vi "RX TX Open (N Channel).vi"(0 "resources":T15[](array[numeric]), 1 "option string":string, 3 "direction":T12, 9 "session in":T1[](array[numeric]), 11 "error in":errorcluster, 12 "force download":bool) -> (4 "tx baseband session out":T2[](array[numeric]), 6 "rx baseband session out":T10[](array[numeric]), 10 "session out":T1[](array[numeric]), 15 "error out":errorcluster)   [LabVIEW 2019] (continued)
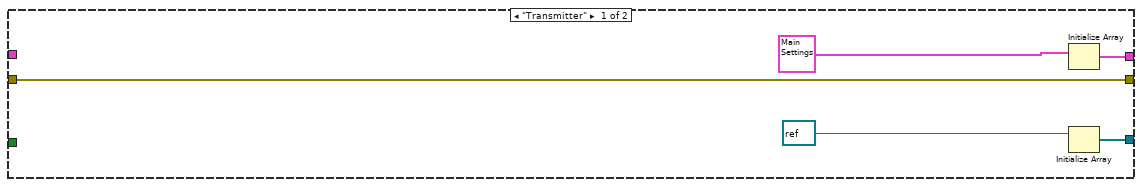
[diagram p2: hidden frame]
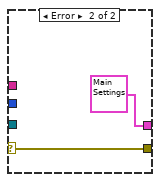
[diagram p4: hidden frame]
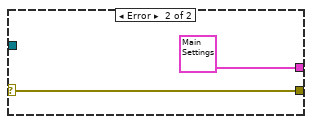
[diagram p5: hidden frame]
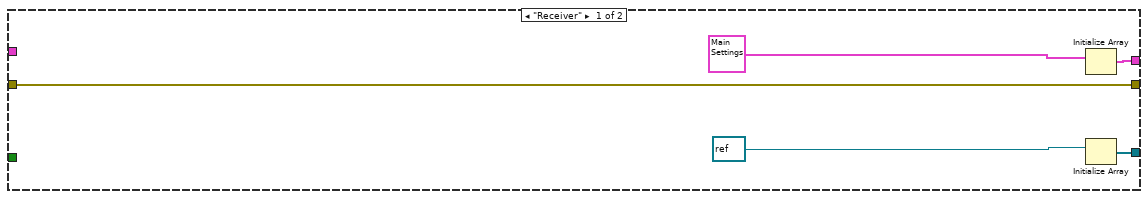
[diagram p6: hidden frame]
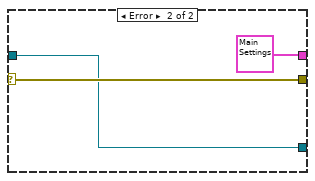
[diagram p7: hidden frame]
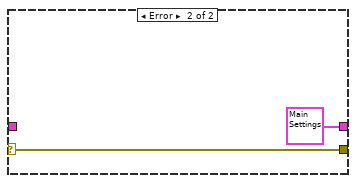
[diagram p10: hidden frame]
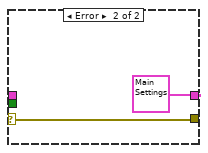
[diagram p12: hidden frame]
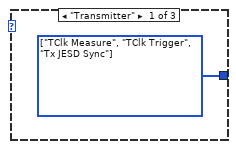
[diagram p13: hidden frame]
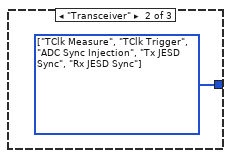
[diagram p14: hidden frame]
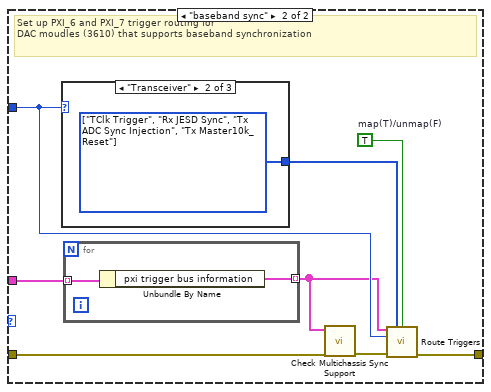
[diagram p15: hidden frame]
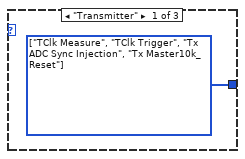
[diagram p16: hidden frame]
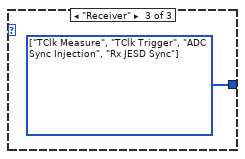
[diagram p17: hidden frame]
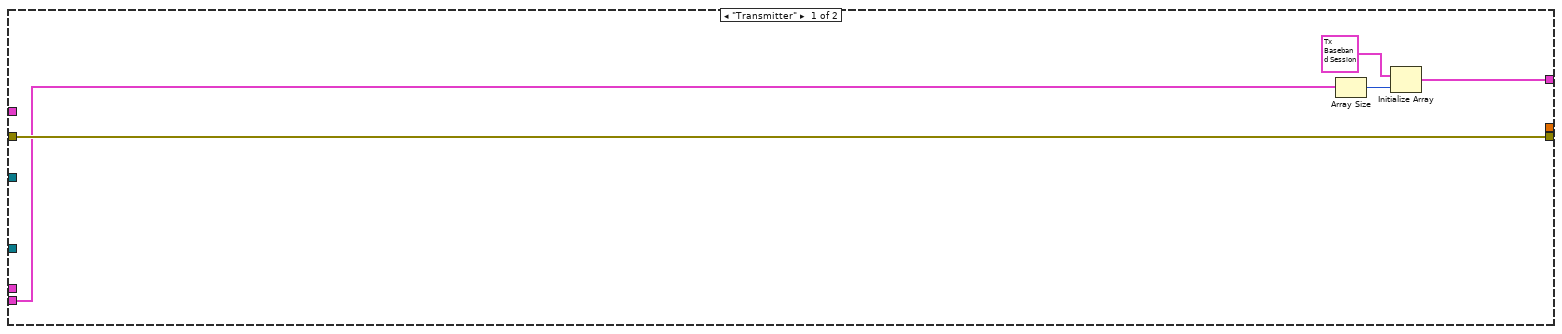
[diagram p18: hidden frame]
          n44 = call "Route Triggers.vi"("pxi trigger bus configuration [channel]"=w230, "route for"=w236, "map(T)/unmap(F)"=w235, "Direction"=w233, "error in"=w231) -> ("error out"=w237:errorcluster)  [unwired: 10 in]
        }
      }
      n45 = case shown="\"Transceiver\", \"Receiver\"" w15 {
        tunnel: w28 -> [w198 w203]
        tunnel: [w197 w202] -> w42
        tunnel: [w198 w201] -> w41
        tunnel: w48 -> [_ w200]
        tunnel: w29 -> [w197 w199]
        frame "Transmitter" {
        }
        frame "Transceiver", "Receiver" {
          n46 = for {
            tunnel: w200 -> [w207]
            shift-right: [w205] -> w202
            shift-left: w199 -> [w208]
            tunnel: w203 -> [w206] mode=indexing
            tunnel: [w204] -> w201 mode=indexing
            # "RX\nInitialize PLL"
            n47 = case shown="No Error" w208 {
              selector: w208 -> [w212 w217]
              tunnel: [w210 w217] -> w205
              tunnel: w206 -> [w213 _]
              tunnel: [w211 T3 {"VISA resource name"=refnum, "Address Space"=0, "window_offset"=0, "register_addresses"={"MM based Registers"={"Revision"=0, "OldestCompatRev"=0, "signature"=0, "scratch"=0, "LedControl"=0, "BoardHwRev"=0, "BoardControl"=0, "ThermalStatus"=0, "BasebandStatus"=0, "BasebandControl"=0, "BasebandAuxSetup"=0, "BasebandAuxStatus"=0, "LmkSyncOutSetup"=0, " AdcSyncOutSetup"=0, " InjSyncOutSetup"=0, " PxiTrig0OutSetup"=0, " PxiTrig1OutSetup"=0, " PxiTrig2OutSetup"=0, " PxiTrig3OutSetup"=0, " PxiTrig4OutSetup"=0, " PxiTrig5OutSetup"=0, " PxiTrig6OutSetup"=0, " PxiTrig7OutSetup"=0}, "CPLD based Registers"={"SlaveSignature"=0, "SlaveRevision"=0, "SlaveOldestCompatRev"=0, "SlaveScratch"=0, "SlaveSetup"=0, "SlaveStatus"=0, "IDacReg_offset"=0, "LMKRegGrp0_offset"=0, "QDacReg_offset"=0, "BrdTempSensorVal"=0, "TempSensorPowerDown"=0, "GPIOReg_offset"=0, "IAdcReg_offset"=0, "QAdcReg_offset"=0, "LMKRegGrp1_offset"=0, "QadcTempSensorVal"=0, "IadcTempSensorVal"=0, "RevisionReg"=0, "VcxoReg"=0, "CpldStatusReg"=0, "PowerReg"=0, "VBiasEnReg"=0, "ExtRefOeReg"=0, "QdacCtrlReg"=0, "QdacStatusReg"=0, "IdacCtrlReg"=0, "IdacStatusReg"=0, "QdacJtagIn"=0, "QdacJtagOut"=0, "IdacJtagIn"=0, "IdacJtagOut"=0, "IqDcSetupReg"=0, "QadcStatusReg"=0, "IadcStatusReg"=0, "BrdSetupReg"=0, "IqDcRevisionReg"=0, "PllStatusReg"=0, "EndpointScratchReg"=0, "AdcSyncCfgReg"=0, "IqCardOpampReg"=0}, "CPLD Register Offset"=0, "MM  Register Offset"=0, " PxiTrig0OutSetup"=0}, "required_MM_fpga_version"={"signature"=0, "hardware"=0, "current revision"=0, "oldest revision"=0}, "CPLD Oldest Compat Version "={"hardware"=0, "CPLD firmware"=0}, "MM_FPGA_image_location"="", "is_init"=FALSE, "card_type"=enum."ADC", "DacLmkConfigFileName"="", "AdcLmkConfigFileName"="", "AdcConfigFileName"="", "DacConfigFileName_RevA"="", "DacConfigFileName_RevB"="", "Mulde hardware revision"=0, "bypass DAC PLL\n"=FALSE, "IQ Card Revision"=enum."RevA", "board capability"={"baseband sync"=enum."no baseband sync"}}] -> w204
              tunnel: w207 -> [w209 _]
              frame No Error {
                # "Combine Initialization Routines"
                n48 = call <instrlib>:"DAC set bypass internal PLL.vi"("error in"=w212, "bypass internal DAC PLL"=w209, "Board Settings in"=w213) -> ("error out"=w215:errorcluster, "Board Settings out"=w214:T3)  [unwired: 7 in]
                n49 = call <instrlib>:"PLL initialize.vi"("error in"=w215, "Board Settings in"=w214) -> ("error out"=w210:errorcluster, "Board Settings out"=w211:T3)  [unwired: 8 in]
              }
              frame Error {
              }
            }
          }
        }
      }
      n50 = case shown="\"Transceiver\", \"Receiver\"" w15 {
        tunnel: w42 -> [w176 w180]
        tunnel: w41 -> [w175 w179]
        tunnel: [w176 w178] -> w37
        tunnel: [w175 w177] -> w38
        frame "Transmitter" {
        }
        frame "Transceiver", "Receiver" {
          n51 = for {
            shift-right: [w184] -> w178
            shift-left: w180 -> [w183]
            tunnel: w179 -> [w182] mode=indexing
            tunnel: [w181] -> w177 mode=indexing
            # "RX\nInitialize ADC"
            n52 = case shown="No Error" w183 {
              selector: w183 -> [w186 w196]
              tunnel: [w188 w196] -> w184
              tunnel: [w189 T3 {"VISA resource name"=refnum, "Address Space"=0, "window_offset"=0, "register_addresses"={"MM based Registers"={"Revision"=0, "OldestCompatRev"=0, "signature"=0, "scratch"=0, "LedControl"=0, "BoardHwRev"=0, "BoardControl"=0, "ThermalStatus"=0, "BasebandStatus"=0, "BasebandControl"=0, "BasebandAuxSetup"=0, "BasebandAuxStatus"=0, "LmkSyncOutSetup"=0, " AdcSyncOutSetup"=0, " InjSyncOutSetup"=0, " PxiTrig0OutSetup"=0, " PxiTrig1OutSetup"=0, " PxiTrig2OutSetup"=0, " PxiTrig3OutSetup"=0, " PxiTrig4OutSetup"=0, " PxiTrig5OutSetup"=0, " PxiTrig6OutSetup"=0, " PxiTrig7OutSetup"=0}, "CPLD based Registers"={"SlaveSignature"=0, "SlaveRevision"=0, "SlaveOldestCompatRev"=0, "SlaveScratch"=0, "SlaveSetup"=0, "SlaveStatus"=0, "IDacReg_offset"=0, "LMKRegGrp0_offset"=0, "QDacReg_offset"=0, "BrdTempSensorVal"=0, "TempSensorPowerDown"=0, "GPIOReg_offset"=0, "IAdcReg_offset"=0, "QAdcReg_offset"=0, "LMKRegGrp1_offset"=0, "QadcTempSensorVal"=0, "IadcTempSensorVal"=0, "RevisionReg"=0, "VcxoReg"=0, "CpldStatusReg"=0, "PowerReg"=0, "VBiasEnReg"=0, "ExtRefOeReg"=0, "QdacCtrlReg"=0, "QdacStatusReg"=0, "IdacCtrlReg"=0, "IdacStatusReg"=0, "QdacJtagIn"=0, "QdacJtagOut"=0, "IdacJtagIn"=0, "IdacJtagOut"=0, "IqDcSetupReg"=0, "QadcStatusReg"=0, "IadcStatusReg"=0, "BrdSetupReg"=0, "IqDcRevisionReg"=0, "PllStatusReg"=0, "EndpointScratchReg"=0, "AdcSyncCfgReg"=0, "IqCardOpampReg"=0}, "CPLD Register Offset"=0, "MM  Register Offset"=0, " PxiTrig0OutSetup"=0}, "required_MM_fpga_version"={"signature"=0, "hardware"=0, "current revision"=0, "oldest revision"=0}, "CPLD Oldest Compat Version "={"hardware"=0, "CPLD firmware"=0}, "MM_FPGA_image_location"="", "is_init"=FALSE, "card_type"=enum."ADC", "DacLmkConfigFileName"="", "AdcLmkConfigFileName"="", "AdcConfigFileName"="", "DacConfigFileName_RevA"="", "DacConfigFileName_RevB"="", "Mulde hardware revision"=0, "bypass DAC PLL\n"=FALSE, "IQ Card Revision"=enum."RevA", "board capability"={"baseband sync"=enum."no baseband sync"}}] -> w181
              tunnel: w182 -> [w185 _]
              frame No Error {
                w187 = T23[] [enum."I-path device", enum."Q-path device"] items=["I-path device", "Q-path device"]
                # "``"
                n53 = for {
                  shift-right: [w192] -> w189
                  shift-left: w185 -> [w194]
                  shift-right: [w191] -> w188
                  shift-left: w186 -> [w193]
                  tunnel: w187 -> [w190] mode=indexing
                  n54 = call <instrlib>:"ADC Initialize.vi"("Board Settings in"=w194, "error in"=w193, "Converter Selection"=w190) -> ("Board Settings out"=w192:T3, "error out"=w191:errorcluster)  [unwired: 6 in]
                }
              }
              frame Error {
              }
            }
          }
        }
      }
      n55 = case shown="\"Transceiver\", \"Receiver\"" w15 {
        selector: w15 -> [_ w250]
        tunnel: [w247 w254] -> w13
        tunnel: [w244 w253] -> w32
        tunnel: w37 -> [w247 w262]
        tunnel: w38 -> [_ w261]
        tunnel: w39 -> [_ w260]
        tunnel: w18 -> [_ w259]
        tunnel: w36 -> [_ w258]
        tunnel: w35 -> [w243 _]
        tunnel: [_ w255] -> w33
        tunnel: w19 -> [_ w252]
        frame "Transmitter" {
          n56 = Array Size(array=w243) -> (size(s)=w246:i32)
          n57 = Initialize Array(T2 {"3610 session"={"VISA resource name"=refnum, "Address Space"=0, "window_offset"=0, "register_addresses"={"MM based Registers"={"Revision"=0, "OldestCompatRev"=0, "signature"=0, "scratch"=0, "LedControl"=0, "BoardHwRev"=0, "BoardControl"=0, "ThermalStatus"=0, "BasebandStatus"=0, "BasebandControl"=0, "BasebandAuxSetup"=0, "BasebandAuxStatus"=0, "LmkSyncOutSetup"=0, " AdcSyncOutSetup"=0, " InjSyncOutSetup"=0, " PxiTrig0OutSetup"=0, " PxiTrig1OutSetup"=0, " PxiTrig2OutSetup"=0, " PxiTrig3OutSetup"=0, " PxiTrig4OutSetup"=0, " PxiTrig5OutSetup"=0, " PxiTrig6OutSetup"=0, " PxiTrig7OutSetup"=0}, "CPLD based Registers"={"SlaveSignature"=0, "SlaveRevision"=0, "SlaveOldestCompatRev"=0, "SlaveScratch"=0, "SlaveSetup"=0, "SlaveStatus"=0, "IDacReg_offset"=0, "LMKRegGrp0_offset"=0, "QDacReg_offset"=0, "BrdTempSensorVal"=0, "TempSensorPowerDown"=0, "GPIOReg_offset"=0, "IAdcReg_offset"=0, "QAdcReg_offset"=0, "LMKRegGrp1_offset"=0, "QadcTempSensorVal"=0, "IadcTempSensorVal"=0, "RevisionReg"=0, "VcxoReg"=0, "CpldStatusReg"=0, "PowerReg"=0, "VBiasEnReg"=0, "ExtRefOeReg"=0, "QdacCtrlReg"=0, "QdacStatusReg"=0, "IdacCtrlReg"=0, "IdacStatusReg"=0, "QdacJtagIn"=0, "QdacJtagOut"=0, "IdacJtagIn"=0, "IdacJtagOut"=0, "IqDcSetupReg"=0, "QadcStatusReg"=0, "IadcStatusReg"=0, "BrdSetupReg"=0, "IqDcRevisionReg"=0, "PllStatusReg"=0, "EndpointScratchReg"=0, "AdcSyncCfgReg"=0, "IqCardOpampReg"=0}, "CPLD Register Offset"=0, "MM  Register Offset"=0, " PxiTrig0OutSetup"=0}, "required_MM_fpga_version"={"signature"=0, "hardware"=0, "current revision"=0, "oldest revision"=0}, "CPLD Oldest Compat Version "={"hardware"=0, "CPLD firmware"=0}, "MM_FPGA_image_location"="", "is_init"=FALSE, "card_type"=enum."ADC", "DacLmkConfigFileName"="", "AdcLmkConfigFileName"="", "AdcConfigFileName"="", "DacConfigFileName_RevA"="", "DacConfigFileName_RevB"="", "Mulde hardware revision"=0, "bypass DAC PLL\n"=FALSE, "IQ Card Revision"=enum."RevA", "board capability"={"baseband sync"=enum."no baseband sync"}}, "7902 reference"=refnum}, w246) -> (w244:T2[])
        }
        frame "Transceiver", "Receiver" {
          n58 = for {
            tunnel: w258 -> [w283] mode=indexing
            shift-right: [w282] -> w256
            shift-left: w262 -> [w268]
            tunnel: [w271] -> w257 mode=indexing
            tunnel: w261 -> [w269] mode=indexing
            tunnel: w260 -> [w270]
            tunnel: w259 -> [w267] mode=indexing
            tunnel: w252 -> [w266]
            tunnel: [w265] -> w251
            tunnel: w250 -> [w264]
            tunnel: [w263] -> w249
            # "RX\nJESD synchronization over PXI_Trig5, apply fractional delay from calibration data and measure ADC relative skew using sync pulse injection on PXI_Trig6"
            n59 = case shown="No Error" w268 {
              selector: w268 -> [w288 w328]
              tunnel: w267 -> [w295 _]
              tunnel: [w292 _] -> w271
              tunnel: [w290 w328] -> w275
              tunnel: w269 -> [w287 _]
              tunnel: w266 -> [w286 w327]
              tunnel: [w286 w327] -> w265
              tunnel: w264 -> [w285 w326]
              tunnel: [w285 w326] -> w263
              frame No Error {
                (unwired) T10 {"3630 session"={"VISA resource name"=refnum, "Address Space"=1, "window_offset"=0, "register_addresses"={"MM based Registers"={"Revision"=0, "OldestCompatRev"=0, "signature"=0, "scratch"=0, "LedControl"=0, "BoardHwRev"=0, "BoardControl"=0, "ThermalStatus"=0, "BasebandStatus"=0, "BasebandControl"=0, "BasebandAuxSetup"=0, "BasebandAuxStatus"=0, "LmkSyncOutSetup"=0, " AdcSyncOutSetup"=0, " InjSyncOutSetup"=0, " PxiTrig0OutSetup"=0, " PxiTrig1OutSetup"=0, " PxiTrig2OutSetup"=0, " PxiTrig3OutSetup"=0, " PxiTrig4OutSetup"=0, " PxiTrig5OutSetup"=0, " PxiTrig6OutSetup"=0, " PxiTrig7OutSetup"=0}, "CPLD based Registers"={"SlaveSignature"=0, "SlaveRevision"=0, "SlaveOldestCompatRev"=0, "SlaveScratch"=0, "SlaveSetup"=0, "SlaveStatus"=0, "IDacReg_offset"=0, "LMKRegGrp0_offset"=0, "QDacReg_offset"=0, "BrdTempSensorVal"=0, "TempSensorPowerDown"=0, "GPIOReg_offset"=0, "IAdcReg_offset"=0, "QAdcReg_offset"=0, "LMKRegGrp1_offset"=0, "QadcTempSensorVal"=0, "IadcTempSensorVal"=0, "RevisionReg"=0, "VcxoReg"=0, "CpldStatusReg"=0, "PowerReg"=0, "VBiasEnReg"=0, "ExtRefOeReg"=0, "QdacCtrlReg"=0, "QdacStatusReg"=0, "IdacCtrlReg"=0, "IdacStatusReg"=0, "QdacJtagIn"=0, "QdacJtagOut"=0, "IdacJtagIn"=0, "IdacJtagOut"=0, "IqDcSetupReg"=0, "QadcStatusReg"=0, "IadcStatusReg"=0, "BrdSetupReg"=0, "IqDcRevisionReg"=0, "PllStatusReg"=0, "EndpointScratchReg"=0, "AdcSyncCfgReg"=0, "IqCardOpampReg"=0}, "CPLD Register Offset"=0, "MM  Register Offset"=0, " PxiTrig0OutSetup"=0}, "required_MM_fpga_version"={"signature"=0, "hardware"=0, "current revision"=0, "oldest revision"=0}, "CPLD Oldest Compat Version "={"hardware"=0, "CPLD firmware"=0}, "MM_FPGA_image_location"="", "is_init"=FALSE, "card_type"=enum."ADC", "DacLmkConfigFileName"="", "AdcLmkConfigFileName"="", "AdcConfigFileName"="", "DacConfigFileName_RevA"="", "DacConfigFileName_RevB"="", "Mulde hardware revision"=0, "bypass DAC PLL\n"=FALSE, "IQ Card Revision"=enum."RevA", "board capability"={"baseband sync"=enum."no baseband sync"}}, "7902 reference"=refnum}
                n60 = call "Enable Reference Output.vi"("Mulde_board_settings_in"=w287, "output reference enable"=FALSE, "error in"=w288) -> ("Mulde_board_settings_out"=w298:T3, "error out"=w300:errorcluster)  [unwired: 11 in]
                n61 = Bundle By Name(cluster=T10 {"3630 session"={"VISA resource name"=refnum, "Address Space"=1, "window_offset"=0, "register_addresses"={"MM based Registers"={"Revision"=0, "OldestCompatRev"=0, "signature"=0, "scratch"=0, "LedControl"=0, "BoardHwRev"=0, "BoardControl"=0, "ThermalStatus"=0, "BasebandStatus"=0, "BasebandControl"=0, "BasebandAuxSetup"=0, "BasebandAuxStatus"=0, "LmkSyncOutSetup"=0, " AdcSyncOutSetup"=0, " InjSyncOutSetup"=0, " PxiTrig0OutSetup"=0, " PxiTrig1OutSetup"=0, " PxiTrig2OutSetup"=0, " PxiTrig3OutSetup"=0, " PxiTrig4OutSetup"=0, " PxiTrig5OutSetup"=0, " PxiTrig6OutSetup"=0, " PxiTrig7OutSetup"=0}, "CPLD based Registers"={"SlaveSignature"=0, "SlaveRevision"=0, "SlaveOldestCompatRev"=0, "SlaveScratch"=0, "SlaveSetup"=0, "SlaveStatus"=0, "IDacReg_offset"=0, "LMKRegGrp0_offset"=0, "QDacReg_offset"=0, "BrdTempSensorVal"=0, "TempSensorPowerDown"=0, "GPIOReg_offset"=0, "IAdcReg_offset"=0, "QAdcReg_offset"=0, "LMKRegGrp1_offset"=0, "QadcTempSensorVal"=0, "IadcTempSensorVal"=0, "RevisionReg"=0, "VcxoReg"=0, "CpldStatusReg"=0, "PowerReg"=0, "VBiasEnReg"=0, "ExtRefOeReg"=0, "QdacCtrlReg"=0, "QdacStatusReg"=0, "IdacCtrlReg"=0, "IdacStatusReg"=0, "QdacJtagIn"=0, "QdacJtagOut"=0, "IdacJtagIn"=0, "IdacJtagOut"=0, "IqDcSetupReg"=0, "QadcStatusReg"=0, "IadcStatusReg"=0, "BrdSetupReg"=0, "IqDcRevisionReg"=0, "PllStatusReg"=0, "EndpointScratchReg"=0, "AdcSyncCfgReg"=0, "IqCardOpampReg"=0}, "CPLD Register Offset"=0, "MM  Register Offset"=0, " PxiTrig0OutSetup"=0}, "required_MM_fpga_version"={"signature"=0, "hardware"=0, "current revision"=0, "oldest revision"=0}, "CPLD Oldest Compat Version "={"hardware"=0, "CPLD firmware"=0}, "MM_FPGA_image_location"="", "is_init"=FALSE, "card_type"=enum."ADC", "DacLmkConfigFileName"="", "AdcLmkConfigFileName"="", "AdcConfigFileName"="", "DacConfigFileName_RevA"="", "DacConfigFileName_RevB"="", "Mulde hardware revision"=0, "bypass DAC PLL\n"=FALSE, "IQ Card Revision"=enum."RevA", "board capability"={"baseband sync"=enum."no baseband sync"}}, "7902 reference"=refnum}, "3630 session"=w298, "7902 reference"=w295) -> (w297:T10)
                n62 = case shown="No Error" w300 {
                  selector: w300 -> [w309 w325]
                  tunnel: [w304 w325] -> w289
                  tunnel: w297 -> [w303 w324]
                  tunnel: [w310 w324] -> w292
                  tunnel: w286 -> [w302 _]
                  tunnel: w285 -> [w301 _]
                  frame No Error {
                    # "JESD synchronizztion on PXI_Trig5"
                    n63 = while {
                      shift-right: [w313] -> w310
                      shift-left: w303 -> [w315]
                      shift-right: [w323] -> w305
                      shift-left: w309 -> [w322]
                      tunnel: [w316] -> w307
                      tunnel: w302 -> [w312]
                      tunnel: w301 -> [w311]
                      i -> [w320]
                      stop <- w317 continue-if-true
                      n64 = call "Configure Chevelle JESD Rx.vi"("rx baseband session in"=w315, "error in"=w322) -> ("rx baseband session"=w314:T10, "error out"=w321:errorcluster)  [unwired: 12 in]
                      n65 = Greater?(x=4, y=w320) -> (0:w318:bool)
                      n66 = call "RX JESD Sync.vi"("rx baseband session in"=w314, "fpga reference in"=w312, "direction"=w311, "error in"=w321) -> ("rx baseband session out"=w313:T10, "timeout error"=w316:bool, "error out"=w323:errorcluster)  [unwired: 9 in]
                      n67 = And(x=w316, y=w318) -> (x .and. y?=w317:bool)
                    }
                    n68 = Merge Errors(w305, errorcluster {"status"=TRUE, "code"=-1, "source"="Could not initialize JESD link"}) -> (w306:errorcluster)
                    n69 = Select(t=w306, s=w307, f=w305) -> (s? t:f=w304:errorcluster)
                  }
                  frame Error {
                  }
                }
                n70 = Unbundle By Name(w292) -> ("7902 reference"=w293:T9)
                n71 = Dynamic FPGA Interface Cast(Session In=T18 refnum, Type=w293) -> (Session Out=w284:T18)
                n72 = call "Configure IQ Inversion.vi"("fpga reference in"=w284, "iq inversion"=cluster{"invert I":bool, "invert Q":bool} {"invert I"=FALSE, "invert Q"=FALSE}, "error in"=w289) -> ("error out"=w290:errorcluster)  [unwired: 11 in, 1 out]
              }
              frame Error {
              }
            }
            n73 = Unbundle By Name(w283) -> ("mulde resource"=w273:refnum<visa-resource-name>)
            n74 = call <instrlib>:"Load Baseband IQ Characterization Data.vi"("VISA resource name"=w273, "error in (no error)"=w275) -> ("Characterization Data"=w281:T24, "error out"=w276:errorcluster)  [unwired: 12 in, 4 out]
            n75 = Unbundle By Name(w281) -> ("Channel Delay"=w279:dbl)
            n76 = Multiply(x=w279, y=1e-12) -> (x*y=w278:dbl)
            n77 = Multiply(x=w278, y=w270) -> (x*y=w277:dbl)
            n78 = Unbundle By Name(w271) -> ("7902 reference"=w272:T9)
            n79 = Negate(x=w277) -> (-x=w274:dbl)
            n80 = call "Set Fractional Delay.vi"("fpga reference in"=w272, "delay (samples)"=w274, "error in"=w276) -> ("error out"=w282:errorcluster)  [unwired: 11 in, 1 out]
          }
          n81 = call "RX Multi Module Sync.vi"("rx baseband session in"=w257, "direction"=w249, "fpga reference in"=w251, "absolute delay"=FALSE, "error in"=w256) -> ("rx baseband session out"=w253:T10[], "measured skew (samples)"=w255:dbl[], "error out"=w254:errorcluster)  [unwired: 8 in]
        }
      }
      n82 = Index Array(array=w21, index=0) -> (element=w14:T3)
      n83 = Unbundle By Name(w14) -> ("board capability.baseband sync"=w17:enum16{"no baseband sync", "baseband sync"})
      n84 = case shown="\"baseband sync\"" w17 {
        tunnel: [w329 w334] -> w44
        tunnel: w18 -> [_ w340]
        tunnel: w19 -> [_ w339]
        tunnel: w21 -> [_ w338]
        tunnel: w13 -> [w329 w331]
        tunnel: w15 -> [_ w332]
        tunnel: w14 -> [_ w333]
        frame "no baseband sync", Default {
        }
        frame "baseband sync" {
          # "Initialize PLL on 3610 modules and perform baseband synchronization using two 10Khz pulses to reset PLL R divider and Sysref counter output"
          n85 = case shown="\"Transceiver\", Default" w332 {
            tunnel: w333 -> [w343 _]
            tunnel: w331 -> [w342 w344]
            tunnel: [w341 w344] -> w330
            frame "Transceiver", Default {
              n86 = call <instrlib>:"PLL initialize.vi"("error in"=w342, "Board Settings in"=w343) -> ("error out"=w341:errorcluster)  [unwired: 8 in, 1 out]
            }
            frame "Receiver" {
            }
          }
          n87 = Build Array (concatenate)(w339, w340) -> (w336:T9[])
          n88 = call "Set 20 kHz TClk Parameters.vi"("fpga reference in"=w336, "error in"=w330) -> ("fpga reference out"=w335:refnum<k20>[], "error out"=w337:errorcluster)  [unwired: 12 in]
          n89 = case shown="\"Transceiver\", \"Transmitter\", Default" w332 {
            tunnel: w338 -> [w348 _]
            tunnel: w337 -> [w347 w349]
            tunnel: w335 -> [w346 _]
            tunnel: [w345 w349] -> w334
            frame "Transceiver", "Transmitter", Default {
              n90 = call "Forward BP Trigger.vi"("fpga reference in"=w346, "Board Settings in"=w348, "error in"=w347) -> ("error out"=w345:errorcluster)  [unwired: 10 in, 2 out]
            }
            frame "Receiver" {
            }
          }
        }
      }
      n91 = case shown="\"baseband sync\"" w17 {
        tunnel: w19 -> [w351 w355]
        tunnel: w18 -> [w352 w354]
        tunnel: [w350 w353] -> w16
        frame "no baseband sync", Default {
          # "Rx 7902 is master"
          n92 = Build Array (concatenate)(w352, w351) -> (w350:T9[])
        }
        frame "baseband sync" {
          # "Tx 7902 is master"
          n93 = Build Array (concatenate)(w355, w354) -> (w353:T9[])
        }
      }
      n94 = flat-sequence {
        tunnel: [w57] -> w40
        tunnel: w44 -> [w70]
        tunnel: w21 -> [w55]
        tunnel: w16 -> [w54]
        frame #0 {
          # "20 kHz TClk as this is a common divider\nfor both 3.072 GHz and 2.94912 GHz"
          # "Align tclk"
          n95 = call "Get Constants.vi"() -> ("constants"=w66:T20)  [unwired: 15 in]
          n96 = Unbundle By Name(w66) -> ("data clock rate (Hz)"=w60:dbl, "sample rate (Hz)"=w64:dbl)
          n97 = for {
            tunnel: [w72] -> w58 mode=indexing if=w73
            tunnel: w54 -> [w72] mode=indexing
            n98 = Not A Number/Path/Refnum?(number/path/refnum=w72) -> (NaN/Path/Refnum?=w74:bool)
            n99 = Not(x=w74) -> (.not. x?=w73:bool)
          }
          n100 = Divide(x=w60, y=20000.0) -> (x/y=w61:dbl)
          n101 = To Unsigned Word Integer(number=w61) -> (unsigned 16bit integer=w62:u16)
          n102 = Bundle By Name(cluster=T17 {"tclk divider"=192, "fpga data clock (Hz)"=192000000.0, "sample rate (Hz)"=3072000000.0}, "tclk divider"=w62, "fpga data clock (Hz)"=w60, "sample rate (Hz)"=w64) -> (w63:T17)
          n103 = call "Set Alignment Complete.vi"("fpga ref in"=w58, "alignment complete"=FALSE, "error in"=w70) -> ("fpga ref out"=w67:T9[], "error out"=w69:errorcluster)  [unwired: 11 in]
          n104 = Array Size(array=w67) -> (size(s)=w71:i32)
          n105 = Initialize Array(w63, w71) -> (w56:T17[])
          n106 = call "Align TClk.vi"("fpga ref in"=w67, "TClk parameters"=w56, "Board Settings in"=w55, "error in"=w69) -> ("error out"=w57:errorcluster)  [unwired: 9 in, 2 out]
        }
      }
      n107 = case shown="\"Transceiver\", \"Transmitter\"" w15 {
        tunnel: w40 -> [w446 w450]
        tunnel: w21 -> [w445 w449]
        tunnel: [w446 w448] -> w31
        tunnel: [w445 w447] -> w30
        frame "Receiver" {
        }
        frame "Transceiver", "Transmitter" {
          n108 = for {
            shift-right: [w452] -> w448
            shift-left: w450 -> [w454]
            tunnel: w449 -> [w453] mode=indexing
            tunnel: [w451] -> w447 mode=indexing
            # "TX\nIntialize PLL"
            n109 = case shown="No Error" w454 {
              selector: w454 -> [w458 w460]
              tunnel: [w457 w460] -> w452
              tunnel: w453 -> [w456 _]
              tunnel: [w455 T3 {"VISA resource name"=refnum, "Address Space"=0, "window_offset"=0, "register_addresses"={"MM based Registers"={"Revision"=0, "OldestCompatRev"=0, "signature"=0, "scratch"=0, "LedControl"=0, "BoardHwRev"=0, "BoardControl"=0, "ThermalStatus"=0, "BasebandStatus"=0, "BasebandControl"=0, "BasebandAuxSetup"=0, "BasebandAuxStatus"=0, "LmkSyncOutSetup"=0, " AdcSyncOutSetup"=0, " InjSyncOutSetup"=0, " PxiTrig0OutSetup"=0, " PxiTrig1OutSetup"=0, " PxiTrig2OutSetup"=0, " PxiTrig3OutSetup"=0, " PxiTrig4OutSetup"=0, " PxiTrig5OutSetup"=0, " PxiTrig6OutSetup"=0, " PxiTrig7OutSetup"=0}, "CPLD based Registers"={"SlaveSignature"=0, "SlaveRevision"=0, "SlaveOldestCompatRev"=0, "SlaveScratch"=0, "SlaveSetup"=0, "SlaveStatus"=0, "IDacReg_offset"=0, "LMKRegGrp0_offset"=0, "QDacReg_offset"=0, "BrdTempSensorVal"=0, "TempSensorPowerDown"=0, "GPIOReg_offset"=0, "IAdcReg_offset"=0, "QAdcReg_offset"=0, "LMKRegGrp1_offset"=0, "QadcTempSensorVal"=0, "IadcTempSensorVal"=0, "RevisionReg"=0, "VcxoReg"=0, "CpldStatusReg"=0, "PowerReg"=0, "VBiasEnReg"=0, "ExtRefOeReg"=0, "QdacCtrlReg"=0, "QdacStatusReg"=0, "IdacCtrlReg"=0, "IdacStatusReg"=0, "QdacJtagIn"=0, "QdacJtagOut"=0, "IdacJtagIn"=0, "IdacJtagOut"=0, "IqDcSetupReg"=0, "QadcStatusReg"=0, "IadcStatusReg"=0, "BrdSetupReg"=0, "IqDcRevisionReg"=0, "PllStatusReg"=0, "EndpointScratchReg"=0, "AdcSyncCfgReg"=0, "IqCardOpampReg"=0}, "CPLD Register Offset"=0, "MM  Register Offset"=0, " PxiTrig0OutSetup"=0}, "required_MM_fpga_version"={"signature"=0, "hardware"=0, "current revision"=0, "oldest revision"=0}, "CPLD Oldest Compat Version "={"hardware"=0, "CPLD firmware"=0}, "MM_FPGA_image_location"="", "is_init"=FALSE, "card_type"=enum."ADC", "DacLmkConfigFileName"="", "AdcLmkConfigFileName"="", "AdcConfigFileName"="", "DacConfigFileName_RevA"="", "DacConfigFileName_RevB"="", "Mulde hardware revision"=0, "bypass DAC PLL\n"=FALSE, "IQ Card Revision"=enum."RevA", "board capability"={"baseband sync"=enum."no baseband sync"}}] -> w451
              frame No Error {
                # "Combine Initialization Routines"
                n110 = call <instrlib>:"PLL initialize.vi"("error in"=w458, "Board Settings in"=w456) -> ("error out"=w457:errorcluster, "Board Settings out"=w455:T3)  [unwired: 8 in]
              }
              frame Error {
              }
            }
          }
        }
      }
      n111 = case shown="\"Transceiver\", \"Transmitter\"" w15 {
        selector: w15 -> [_ w366]
        tunnel: w31 -> [w360 w378]
        tunnel: w35 -> [_ w377]
        tunnel: w19 -> [_ w376]
        tunnel: w30 -> [_ w374]
        tunnel: [w360 w371] -> w34
        tunnel: w39 -> [_ w370]
        tunnel: [w357 w369] -> w49
        tunnel: w36 -> [w356 _]
        tunnel: w20 -> [_ w365]
        frame "Receiver" {
          n112 = Array Size(array=w356) -> (size(s)=w359:i32)
          n113 = Initialize Array(T2 {"3610 session"={"VISA resource name"=refnum, "Address Space"=0, "window_offset"=0, "register_addresses"={"MM based Registers"={"Revision"=0, "OldestCompatRev"=0, "signature"=0, "scratch"=0, "LedControl"=0, "BoardHwRev"=0, "BoardControl"=0, "ThermalStatus"=0, "BasebandStatus"=0, "BasebandControl"=0, "BasebandAuxSetup"=0, "BasebandAuxStatus"=0, "LmkSyncOutSetup"=0, " AdcSyncOutSetup"=0, " InjSyncOutSetup"=0, " PxiTrig0OutSetup"=0, " PxiTrig1OutSetup"=0, " PxiTrig2OutSetup"=0, " PxiTrig3OutSetup"=0, " PxiTrig4OutSetup"=0, " PxiTrig5OutSetup"=0, " PxiTrig6OutSetup"=0, " PxiTrig7OutSetup"=0}, "CPLD based Registers"={"SlaveSignature"=0, "SlaveRevision"=0, "SlaveOldestCompatRev"=0, "SlaveScratch"=0, "SlaveSetup"=0, "SlaveStatus"=0, "IDacReg_offset"=0, "LMKRegGrp0_offset"=0, "QDacReg_offset"=0, "BrdTempSensorVal"=0, "TempSensorPowerDown"=0, "GPIOReg_offset"=0, "IAdcReg_offset"=0, "QAdcReg_offset"=0, "LMKRegGrp1_offset"=0, "QadcTempSensorVal"=0, "IadcTempSensorVal"=0, "RevisionReg"=0, "VcxoReg"=0, "CpldStatusReg"=0, "PowerReg"=0, "VBiasEnReg"=0, "ExtRefOeReg"=0, "QdacCtrlReg"=0, "QdacStatusReg"=0, "IdacCtrlReg"=0, "IdacStatusReg"=0, "QdacJtagIn"=0, "QdacJtagOut"=0, "IdacJtagIn"=0, "IdacJtagOut"=0, "IqDcSetupReg"=0, "QadcStatusReg"=0, "IadcStatusReg"=0, "BrdSetupReg"=0, "IqDcRevisionReg"=0, "PllStatusReg"=0, "EndpointScratchReg"=0, "AdcSyncCfgReg"=0, "IqCardOpampReg"=0}, "CPLD Register Offset"=0, "MM  Register Offset"=0, " PxiTrig0OutSetup"=0}, "required_MM_fpga_version"={"signature"=0, "hardware"=0, "current revision"=0, "oldest revision"=0}, "CPLD Oldest Compat Version "={"hardware"=0, "CPLD firmware"=0}, "MM_FPGA_image_location"="", "is_init"=FALSE, "card_type"=enum."ADC", "DacLmkConfigFileName"="", "AdcLmkConfigFileName"="", "AdcConfigFileName"="", "DacConfigFileName_RevA"="", "DacConfigFileName_RevB"="", "Mulde hardware revision"=0, "bypass DAC PLL\n"=FALSE, "IQ Card Revision"=enum."RevA", "board capability"={"baseband sync"=enum."no baseband sync"}}, "7902 reference"=refnum}, w359) -> (w357:T2[])
        }
        frame "Transceiver", "Transmitter" {
          n114 = for {
            shift-right: [w398] -> w375
            shift-left: w378 -> [w397]
            tunnel: w370 -> [w396]
            tunnel: w377 -> [w394] mode=indexing
            tunnel: w376 -> [w393] mode=indexing
            tunnel: [w392] -> w373 mode=indexing
            # "TX\napply channel fractional delay"
            n115 = Unbundle By Name(w394) -> ("mulde resource"=w395:refnum<visa-resource-name>)
            n116 = call <instrlib>:"Load Baseband IQ Characterization Data.vi"("VISA resource name"=w395, "error in (no error)"=w397) -> ("Characterization Data"=w401:T24, "error out"=w400:errorcluster)  [unwired: 12 in, 4 out]
            n117 = Unbundle By Name(w401) -> ("Channel Delay"=w399:dbl)
            n118 = Multiply(x=w399, y=1e-12) -> (x*y=w403:dbl)
            n119 = Multiply(x=w403, y=w396) -> (x*y=w404:dbl)
            n120 = Negate(x=w404) -> (-x=w405:dbl)
            n121 = call "Set Fractional Delay.vi"("fpga reference in"=w393, "delay (samples)"=w405, "error in"=w400) -> ("fpga reference out"=w392:T9, "error out"=w398:errorcluster)  [unwired: 11 in]
          }
          n122 = call "Sync SysRef.vi"("fpga reference in"=w373, "board settings in"=w374, "error in"=w375) -> ("fpga reference out"=w372:T9[], "board settings out"=w364:T3[], "error out"=w368:errorcluster)  [unwired: 10 in]
          n123 = Index Array(array=w364, index=0) -> (element=w362:T3)
          n124 = Unbundle By Name(w362) -> ("board capability.baseband sync"=w361:enum16{"no baseband sync", "baseband sync"})
          n125 = case shown="\"baseband sync\"" w361 {
            tunnel: [w379 w386] -> w367
            tunnel: w366 -> [_ w381]
            tunnel: w368 -> [w379 w380]
            tunnel: w365 -> [_ w383]
            frame "no baseband sync", Default {
            }
            frame "baseband sync" {
              w384 = TRUE  # map(T)/unmap(F)
              # "Baseband synchronization on DAC moudles (3610) rev. F or later \nis complete. Revert PXI_7 routing back to Tx JESD sync"
              n126 = case shown="\"Transmitter\"" w381 {
                tunnel: [w389 w390 w391] -> w385
                frame "Transmitter" {
                  w389 = T22 [enum."TClk Measure", enum."TClk Trigger", enum."Tx ADC Sync Injection", enum."Tx JESD Sync"] items=["TClk Trigger", "TClk Measure", "ADC Sync Injection", "Tx JESD Sync", "Rx JESD Sync", "Tx ADC Sync Injection", "Tx Master10k_Reset"]
                }
                frame "Transceiver" {
                  w390 = T22 [enum."TClk Trigger", enum."Rx JESD Sync", enum."Tx ADC Sync Injection", enum."Tx JESD Sync"] items=["TClk Trigger", "TClk Measure", "ADC Sync Injection", "Tx JESD Sync", "Rx JESD Sync", "Tx ADC Sync Injection", "Tx Master10k_Reset"]
                }
                frame "Receiver" {
                  w391 = T22 [enum."TClk Measure", enum."TClk Trigger", enum."ADC Sync Injection", enum."Rx JESD Sync"] items=["TClk Trigger", "TClk Measure", "ADC Sync Injection", "Tx JESD Sync", "Rx JESD Sync", "Tx ADC Sync Injection", "Tx Master10k_Reset"]
                }
              }
              n127 = for {
                tunnel: w383 -> [w388] mode=indexing
                tunnel: [w387] -> w382 mode=indexing
                n128 = Unbundle By Name(w388) -> ("pxi trigger bus information"=w387:T14)
              }
              n129 = call "Route Triggers.vi"("pxi trigger bus configuration [channel]"=w382, "route for"=w385, "map(T)/unmap(F)"=w384, "Direction"=w381, "error in"=w380) -> ("error out"=w386:errorcluster)  [unwired: 10 in]
            }
          }
          n130 = for {
            shift-right: [w415] -> w371
            shift-left: w367 -> [w432]
            tunnel: w372 -> [w408] mode=indexing
            tunnel: w364 -> [w430] mode=indexing
            tunnel: [w409] -> w369 mode=indexing
            w426 = T23[] [enum."I-path device", enum."Q-path device"] items=["I-path device", "Q-path device"]
            w433 = T23[] [enum."I-path device", enum."Q-path device"] items=["I-path device", "Q-path device"]
            # "TX\nInitialize DAC and perform JESD synchronization"
            n131 = for {
              shift-right: [w441] -> w429
              shift-left: w430 -> [w444]
              shift-right: [w440] -> w407
              shift-left: w432 -> [w443]
              tunnel: w433 -> [w442] mode=indexing
              n132 = call <instrlib>:"DAC Initialize.vi"("Board Settings in"=w444, "error in"=w443, "Converter Path Selection"=w442) -> ("Board Settings out"=w441:T3, "error out"=w440:errorcluster)  [unwired: 6 in]
            }
            n133 = call "JESD Sync TX.vi"("fpga ref in"=w408, "txjesd.LmfcDly"=fxp<+,5,5> 1.0, "Board Settings in"=w429, "error in (no error)"=w407) -> ("fpga ref out"=w425:T9, "Board Settings out"=w427:T3, "error out"=w428:errorcluster)  [unwired: 9 in]
            n134 = for {
              shift-right: [w438] -> w419
              shift-left: w428 -> [w439]
              shift-right: [w436] -> w411
              shift-left: w427 -> [w437]
              tunnel: w426 -> [w435] mode=indexing
              n135 = call <instrlib>:"DAC get Alarms.vi"("Board Settings in"=w437, "clear alarms"=TRUE, "Converter Path Selection"=w435, "error in"=w439) -> ("Board Settings out"=w436:T3, "error out"=w438:errorcluster)  [unwired: 13 in, 9 out]
            }
            n136 = Dynamic FPGA Interface Cast(Session In=T19 refnum, Type=w425) -> (Session Out=w421:T19)
            n137 = xnode "Read/Write Control"("FPGA VI Reference In"=w421, "error in"=w419) -> ("FPGA VI Reference Out"=w420:T19, "error out"=w418:errorcluster, "txjesd.control"=w406:T25)
            n138 = Bundle By Name(cluster=w406, "clear data in error"=TRUE) -> (w422:T25)
            n139 = Bundle By Name(cluster=w406, "clear data in error"=FALSE) -> (w414:T25)
            n140 = xnode "Read/Write Control"("FPGA VI Reference In"=w420, "error in"=w418, "txjesd.control"=w422) -> ("FPGA VI Reference Out"=w417:T19, "error out"=w416:errorcluster)
            n141 = xnode "Read/Write Control"("FPGA VI Reference In"=w417, "error in"=w416, "txjesd.control"=w414) -> ("FPGA VI Reference Out"=w410:T19, "error out"=w415:errorcluster)
            n142 = Bundle By Name(cluster=T2 {"3610 session"={"VISA resource name"=refnum, "Address Space"=1, "window_offset"=0, "register_addresses"={"MM based Registers"={"Revision"=0, "OldestCompatRev"=0, "signature"=0, "scratch"=0, "LedControl"=0, "BoardHwRev"=0, "BoardControl"=0, "ThermalStatus"=0, "BasebandStatus"=0, "BasebandControl"=0, "BasebandAuxSetup"=0, "BasebandAuxStatus"=0, "LmkSyncOutSetup"=0, " AdcSyncOutSetup"=0, " InjSyncOutSetup"=0, " PxiTrig0OutSetup"=0, " PxiTrig1OutSetup"=0, " PxiTrig2OutSetup"=0, " PxiTrig3OutSetup"=0, " PxiTrig4OutSetup"=0, " PxiTrig5OutSetup"=0, " PxiTrig6OutSetup"=0, " PxiTrig7OutSetup"=0}, "CPLD based Registers"={"SlaveSignature"=0, "SlaveRevision"=0, "SlaveOldestCompatRev"=0, "SlaveScratch"=0, "SlaveSetup"=0, "SlaveStatus"=0, "IDacReg_offset"=0, "LMKRegGrp0_offset"=0, "QDacReg_offset"=0, "BrdTempSensorVal"=0, "TempSensorPowerDown"=0, "GPIOReg_offset"=0, "IAdcReg_offset"=0, "QAdcReg_offset"=0, "LMKRegGrp1_offset"=0, "QadcTempSensorVal"=0, "IadcTempSensorVal"=0, "RevisionReg"=0, "VcxoReg"=0, "CpldStatusReg"=0, "PowerReg"=0, "VBiasEnReg"=0, "ExtRefOeReg"=0, "QdacCtrlReg"=0, "QdacStatusReg"=0, "IdacCtrlReg"=0, "IdacStatusReg"=0, "QdacJtagIn"=0, "QdacJtagOut"=0, "IdacJtagIn"=0, "IdacJtagOut"=0, "IqDcSetupReg"=0, "QadcStatusReg"=0, "IadcStatusReg"=0, "BrdSetupReg"=0, "IqDcRevisionReg"=0, "PllStatusReg"=0, "EndpointScratchReg"=0, "AdcSyncCfgReg"=0, "IqCardOpampReg"=0}, "CPLD Register Offset"=0, "MM  Register Offset"=0, " PxiTrig0OutSetup"=0}, "required_MM_fpga_version"={"signature"=0, "hardware"=0, "current revision"=0, "oldest revision"=0}, "CPLD Oldest Compat Version "={"hardware"=0, "CPLD firmware"=0}, "MM_FPGA_image_location"="", "is_init"=FALSE, "card_type"=enum."ADC", "DacLmkConfigFileName"="", "AdcLmkConfigFileName"="", "AdcConfigFileName"="", "DacConfigFileName_RevA"="", "DacConfigFileName_RevB"="", "Mulde hardware revision"=0, "bypass DAC PLL\n"=FALSE, "IQ Card Revision"=enum."RevA", "board capability"={"baseband sync"=enum."no baseband sync"}}, "7902 reference"=refnum}, "3610 session"=w411, "7902 reference"=w410) -> (w409:T2)
          }
        }
      }
    }
    frame Error {
    }
  }
  "tx baseband session out" <- w8
  "measured skew (samples)" <- w7
  "rx baseband session out" <- w6
  "error out" <- w9
  "session out" <- w1
